vi "TLB Native Dynamic Events ver 0.26a.vi"() -> ()   [LabVIEW 2018] (continued)
          tunnel: w296 -> [_ _ _ _ _ _ _ _ _ _ _ _ _ _ _ _ _ _ _ _ _ _ _ _ _ _ _ _ _ _ _ _ _ _ _ _ _ _ _ _ w2086 _ _ _ _ _ _ _ w2455 _ _ _ _ _ _]
          tunnel: w295 -> [_ _ _ _ _ w505 _ _ _ _ _ _ _ _ w926 _ _ _ _ _ _ _ _ _ _ _ _ _ _ _ _ _ _ _ _ _ _ _ _ w2036 _ w2130 _ _ w2265 _ _ _ _ w2501 _ _ w2633 _ _]
          tunnel: [w337 w343 w360 w373 w492 w507 w552 w594 w640 w688 w734 w777 w823 w871 w927 w979 w1026 w1072 w1115 w1159 w1208 w1254 w1298 w1344 w1387 w1428 w1434 w1480 w1529 w1573 w1617 w1670 w1714 w1758 w1807 w1853 w1897 w1943 w1988 w2035 w2085 w2131 w2175 w2219 w2277 w2321 w2365 w2411 w2468 w2512 w2556 w2600 w2648 w2692 w2736] -> w293
          tunnel: w292 -> [w337 w343 w360 _ w492 w507 w552 w594 w640 w688 w734 w777 w823 w871 w927 w979 w1026 w1072 w1115 w1159 w1208 w1254 w1298 w1344 w1387 w1428 w1434 w1480 w1529 w1573 w1617 w1670 w1714 w1758 w1807 w1853 w1897 w1943 w1988 w2035 w2085 w2131 w2175 w2219 w2277 w2321 w2365 w2411 w2468 w2512 w2556 w2600 w2648 w2692 w2736]
          tunnel: w291 -> [_ _ _ _ _ _ _ _ _ _ _ _ _ _ _ _ _ _ _ _ _ _ _ _ _ _ _ _ _ _ _ _ _ _ _ _ _ _ _ _ w2084 _ _ _ _ _ _ _ _ _ _ _ _ _ _]
          tunnel: [_ _ _ _ _ _ _ _ w639 _ _ _ _ _ _ _ _ _ _ _ _ _ _ _ _ _ _ _ _ _ _ _ _ _ _ _ _ _ _ _ _ _ _ _ _ _ _ _ w2444 _ _ _ _ _ _] -> w290
          tunnel: [_ _ _ _ _ _ _ _ _ _ _ _ _ _ _ _ _ _ _ _ _ _ _ _ _ _ _ _ _ _ _ _ _ _ _ _ _ _ _ _ w2082 _ _ _ _ _ _ _ _ _ _ _ _ _ _] -> w289
          tunnel: [_ _ _ _ _ _ _ _ _ _ _ _ _ _ _ _ _ _ _ _ _ _ _ _ _ _ _ _ _ _ _ _ _ _ _ _ _ _ _ _ w2081 _ _ _ _ _ _ _ _ _ _ _ _ _ _] -> w288
          tunnel: w287 -> [_ _ _ _ _ _ _ _ _ _ _ _ _ _ _ _ _ _ _ _ _ _ _ _ _ _ _ _ _ _ _ _ _ _ _ _ _ _ _ _ _ _ _ _ _ _ _ _ _ _ _ _ _ _ _]
          frame 0 {
            # ">>> yStepper command>>>"
          }
          frame 1 {
            # ">>> yStepper command>>>"
            n201 = for {
              shift-right: [w359] -> w353
              shift-left: w356 -> [w358]
              tunnel: string[] ["INIT", "RESET ARM", "RESET FLAGS", "RESET YAW", "NAVX CALIBRATE"] -> [w357] mode=indexing
              n202 = Enqueue Element(queue=w358, element=w357) -> (queue out=w359:refnum<queue>)  [unwired: 2 in, 2 out]
            }
            n203 = Bundle By Name(cluster=w351, "yStepper desired"=u8 0) -> (w350:T20)
            n204 = Bundle By Name(cluster=w348, "ySpeed"=0.0, "xSpeed"=0.0, "wSpeed"=0.0) -> (w347:T19)
          }
          frame 3 {
            # ">>Action Queue>>"
            # ">>> Motor control cluster >>>"
            # ">>> yStepper command>>>"
            n205 = Flush Queue(queue=w366, error in (no error)=w365) -> ()  [unwired: 3 out]
            n206 = for {
              shift-right: [w372] -> w367
              shift-left: w368 -> [w371]
              tunnel: string[] ["STOP", "RESET ENCODERS", "RESET YAW", "RESET ARM", "RESET ALL SENSORS", "DISPOSE CAM BUFFERS", "DISPOSE PROC BUFFERS", "CAM CLOSE", ""] -> [w370] mode=indexing
              n207 = Enqueue Element(queue=w371, element=w370) -> (queue out=w372:refnum<queue>)  [unwired: 2 in, 2 out]
            }
          }
          frame 4, Default {
            # ">>> Motor control cluster >>>"
            # ">>> yStepper command>>>"
            n208 = Dequeue Element(queue=w384, timeout in ms (-1)=w383, error in (no error)=w379) -> (element=w382:T10)  [unwired: 3 out]
            n209 = case shown="\"Start Task 9\"" w382 {
              tunnel: [w387 w395 w403 w411 w419 w427 w435 w443 w451 w458 w468 w476 w483 w486] -> w378
              tunnel: w381 -> [w388 w396 w404 w412 w420 w428 w436 w444 w452 w459 w467 w475 w483 w487]
              tunnel: [State_Type_Definitions,_for_0.26g_versions_and_later_2."Task 1A" ("Enum") State_Type_Definitions,_for_0.26g_versions_and_later_2."Task 2:Raise Arm" ("Enum") State_Type_Definitions,_for_0.26g_versions_and_later_2."Task 3" ("Enum") State_Type_Definitions,_for_0.26g_versions_and_later_2."Task 4_A" ("Enum") State_Type_Definitions,_for_0.26g_versions_and_later_2."Task 5A" ("Enum") State_Type_Definitions,_for_0.26g_versions_and_later_2."Task 6_A" ("Enum") State_Type_Definitions,_for_0.26g_versions_and_later_2."Task 8A: RAISE ARM" ("Enum") State_Type_Definitions,_for_0.26g_versions_and_later_2."Task 8A: RAISE ARM" ("Enum") State_Type_Definitions,_for_0.26g_versions_and_later_2."Task 8A: RAISE ARM" ("Enum") State_Type_Definitions,_for_0.26g_versions_and_later_2."Task 8A: RAISE ARM" ("Enum") State_Type_Definitions,_for_0.26g_versions_and_later_2."Task 9A: Raise Arm" ("Enum") State_Type_Definitions."Task 9F: SCAN IMAGE" ("Enum") State_Type_Definitions,_for_0.26g_versions_and_later_2."Idle" ("Enum") State_Type_Definitions,_for_0.26g_versions_and_later_2."Shutdown" ("Enum")] -> w380
              tunnel: [enum16{"Ball", "Soap", "Gel", "Pipe", "None"}."None" ("Object recognition mode") enum16{"Ball", "Soap", "Gel", "Pipe", "None"}."None" ("Object recognition mode") enum16{"Ball", "Soap", "Gel", "Pipe", "None"}."None" ("Object recognition mode") enum16{"Ball", "Soap", "Gel", "Pipe", "None"}."None" ("Object recognition mode") enum16{"Ball", "Soap", "Gel", "Pipe", "None"}."None" ("Object recognition mode") enum16{"Ball", "Soap", "Gel", "Pipe", "None"}."None" ("Object recognition mode") enum16{"Ball", "Soap", "Gel", "Pipe", "None"}."Ball" ("Object recognition mode") enum16{"Ball", "Soap", "Gel", "Pipe", "None"}."Gel" ("Object recognition mode") enum16{"Ball", "Soap", "Gel", "Pipe", "None"}."Pipe" ("Object recognition mode") enum16{"Ball", "Soap", "Gel", "Pipe", "None"}."Soap" ("Object recognition mode") enum16{"Ball", "Soap", "Gel", "Pipe", "None"}."None" ("Object recognition mode") enum16{"Ball", "Soap", "Gel", "Pipe", "None"}."None" ("Object recognition mode") enum16{"Ball", "Soap", "Gel", "Pipe", "None"}."None" ("Object recognition mode") enum16{"Ball", "Soap", "Gel", "Pipe", "None"}."None" ("Object recognition mode")] -> w373
              frame "Start Task 1" {
                n210 = for {
                  shift-right: [w392] -> w387
                  shift-left: w388 -> [w391]
                  tunnel: string[] ["RESET ENCODERS", "RESET YAW", "FORWARD", "READ ENCODERS"] -> [w390] mode=indexing
                  n211 = Enqueue Element(queue=w391, element=w390) -> (queue out=w392:refnum<queue>)  [unwired: 2 in, 2 out]
                }
              }
              frame "Start Task 2" {
                n212 = for {
                  shift-right: [w400] -> w395
                  shift-left: w396 -> [w399]
                  tunnel: string[] ["RESET ENCODERS", "RESET YAW", "READ ULTRASONIC", "ARDUINO - ULTRASONIC"] -> [w398] mode=indexing
                  n213 = Enqueue Element(queue=w399, element=w398) -> (queue out=w400:refnum<queue>)  [unwired: 2 in, 2 out]
                }
              }
              frame "Start Task 3" {
                n214 = for {
                  shift-right: [w408] -> w403
                  shift-left: w404 -> [w407]
                  tunnel: string[] ["RESET ENCODERS", "READ ENCODERS", "R-ACW"] -> [w406] mode=indexing
                  n215 = Enqueue Element(queue=w407, element=w406) -> (queue out=w408:refnum<queue>)  [unwired: 2 in, 2 out]
                }
              }
              frame "Start Task 4" {
                n216 = for {
                  shift-right: [w416] -> w411
                  shift-left: w412 -> [w415]
                  tunnel: string[] ["RESET YAW", "RESET ENCODERS", "RESET ARM", "RESET FLAGS", "", ""] -> [w414] mode=indexing
                  n217 = Enqueue Element(queue=w415, element=w414) -> (queue out=w416:refnum<queue>)  [unwired: 2 in, 2 out]
                }
              }
              frame "Start Task 5" {
                n218 = for {
                  shift-right: [w424] -> w419
                  shift-left: w420 -> [w423]
                  tunnel: string[] ["RESET YAW", "RESET ENCODERS", "RESET ARM", "RESET ALL SENSORS", "", ""] -> [w422] mode=indexing
                  n219 = Enqueue Element(queue=w423, element=w422) -> (queue out=w424:refnum<queue>)  [unwired: 2 in, 2 out]
                }
              }
              frame "Start Task 6" {
                n220 = for {
                  shift-right: [w432] -> w427
                  shift-left: w428 -> [w431]
                  tunnel: string[] ["OPEN LOG CAM ", "", "", "", "", ""] -> [w430] mode=indexing
                  n221 = Enqueue Element(queue=w431, element=w430) -> (queue out=w432:refnum<queue>)  [unwired: 2 in, 2 out]
                }
              }
              frame "Start Task 8 - BALL" {
                n222 = for {
                  shift-right: [w440] -> w435
                  shift-left: w436 -> [w439]
                  tunnel: string[] ["RESET YAW", "RESET ENCODERS", "RESET ARM", "RESET FLAGS"] -> [w438] mode=indexing
                  n223 = Enqueue Element(queue=w439, element=w438) -> (queue out=w440:refnum<queue>)  [unwired: 2 in, 2 out]
                }
              }
              frame "Start Task 8 - Gel" {
                n224 = for {
                  shift-right: [w448] -> w443
                  shift-left: w444 -> [w447]
                  tunnel: string[] ["RESET YAW", "RESET ENCODERS", "RESET ARM", "RESET FLAGS"] -> [w446] mode=indexing
                  n225 = Enqueue Element(queue=w447, element=w446) -> (queue out=w448:refnum<queue>)  [unwired: 2 in, 2 out]
                }
              }
              frame "Start Task 8 - Pipe" {
                n226 = for {
                  shift-right: [w456] -> w451
                  shift-left: w452 -> [w455]
                  tunnel: string[] ["RESET YAW", "RESET ENCODERS", "RESET ARM", "RESET FLAGS"] -> [w454] mode=indexing
                  n227 = Enqueue Element(queue=w455, element=w454) -> (queue out=w456:refnum<queue>)  [unwired: 2 in, 2 out]
                }
              }
              frame "Start Task 8 - Soap" {
                n228 = for {
                  shift-right: [w464] -> w458
                  shift-left: w459 -> [w463]
                  tunnel: string[] ["RESET YAW", "RESET ENCODERS", "RESET ARM", "RESET FLAGS"] -> [w462] mode=indexing
                  n229 = Enqueue Element(queue=w463, element=w462) -> (queue out=w464:refnum<queue>)  [unwired: 2 in, 2 out]
                }
              }
              frame "Start Task 9" {
                n230 = for {
                  shift-right: [w472] -> w468
                  shift-left: w467 -> [w471]
                  tunnel: string[] ["RESET ENCODERS", "READ ENCODERS", "Z STEPPER BOX HEIGHT"] -> [w470] mode=indexing
                  n231 = Enqueue Element(queue=w471, element=w470) -> (queue out=w472:refnum<queue>)  [unwired: 2 in, 2 out]
                }
              }
              frame "Start Task A" {
                n232 = for {
                  shift-right: [w480] -> w476
                  shift-left: w475 -> [w479]
                  tunnel: string[] ["RESET ENCODERS", "READ ENCODERS", "RESET YAW", "Z STEPPER BOX HEIGHT"] -> [w478] mode=indexing
                  n233 = Enqueue Element(queue=w479, element=w478) -> (queue out=w480:refnum<queue>)  [unwired: 2 in, 2 out]
                }
              }
              frame "None", Default {
              }
              frame "Exit" {
                n234 = for {
                  shift-right: [w491] -> w486
                  shift-left: w487 -> [w490]
                  tunnel: string[] ["STOP", "RESET ENCODERS", "RESET YAW", "EXIT"] -> [w489] mode=indexing
                  n235 = Enqueue Element(queue=w490, element=w489) -> (queue out=w491:refnum<queue>)  [unwired: 2 in, 2 out]
                }
              }
            }
          }
          frame 5 {
            # ">> Item Selection Bias >>"
            # ">>> yStepper command>>>"
            n236 = for {
              shift-right: [w502] -> w496
              shift-left: w498 -> [w501]
              tunnel: string[] ["INIT", "RESET ENCODERS", "RESET FLAGS", "CAM CLOSE", "DISPOSE BUFFERS", "EXIT", ""] -> [w500] mode=indexing
              n237 = Enqueue Element(queue=w501, element=w500) -> (queue out=w502:refnum<queue>)  [unwired: 2 in, 2 out]
            }
          }
          frame 6 {
            # ">>> Motor control cluster >>>"
            # ">> Line detection >>"
            # ">> Checks if 1 metre moved >>"
            # ">>> yStepper command>>>"
            # "Use 250"
            n238 = Greater?(x=w512, y=265.0) -> (0:w506:bool)
            n239 = Dequeue Element(queue=w519, timeout in ms (-1)=w518, error in (no error)=w517) -> (element=w516:T10)  [unwired: 3 out]
            n240 = And(x=w505, y=w506) -> (x .and. y?=w503:bool)
            n241 = case shown="\"Start Task 1\", Default" w516 {
              tunnel: w504 -> [w520 _]
              tunnel: [w530 State_Type_Definitions,_for_0.26g_versions_and_later_2."True Stop" ("Enum")] -> w515
              tunnel: w514 -> [w528 w545]
              tunnel: [w527 w544] -> w513
              tunnel: [State_Type_Definitions,_for_0.26g_versions_and_later_2."Idle" ("Enum") State_Type_Definitions,_for_0.26g_versions_and_later_2."Shutdown" ("Enum")] -> w510
              tunnel: w503 -> [w521 _]
              frame "Start Task 1", Default {
                n242 = Or(x=w521, y=w520) -> (x .or. y?=w522:bool)
                n243 = case shown="True" w522 {
                  tunnel: w528 -> [w533 w539]
                  tunnel: [w532 w537] -> w527
                  frame False {
                    n244 = for {
                      shift-right: [w535] -> w532
                      shift-left: w533 -> [w536]
                      tunnel: string[] ["READ ENCODERS", "READ NAVX", "FORWARD", "READ LINE SENSOR"] ("element") -> [w534] mode=indexing
                      n245 = Enqueue Element(queue=w536, element=w534) -> (queue out=w535:refnum<queue>)  [unwired: 2 in, 2 out]
                    }
                  }
                  frame True {
                    n246 = for {
                      shift-right: [w541] -> w537
                      shift-left: w539 -> [w542]
                      tunnel: string[] ["RESET YAW", "RESET ENCODERS", "STOP", ""] -> [w540] mode=indexing
                      n247 = Enqueue Element(queue=w542, element=w540) -> (queue out=w541:refnum<queue>)  [unwired: 2 in, 2 out]
                    }
                  }
                }
                n248 = Select(t=State_Type_Definitions,_for_0.26g_versions_and_later_2."True Stop" ("Enum"), s=w520, f=State_Type_Definitions,_for_0.26g_versions_and_later_2."Task 1B" ("Enum")) -> (s? t:f=w525:T18)
                n249 = Select(t=w525, s=w521, f=State_Type_Definitions,_for_0.26g_versions_and_later_2."Task 1A" ("Enum")) -> (s? t:f=w530:T18)
              }
              frame "Exit" {
                n250 = for {
                  shift-right: [w549] -> w544
                  shift-left: w545 -> [w550]
                  tunnel: string[] ["STOP", "RESET ENCODERS", "RESET YAW", ""] -> [w548] mode=indexing
                  n251 = Enqueue Element(queue=w550, element=w548) -> (queue out=w549:refnum<queue>)  [unwired: 2 in, 2 out]
                }
              }
            }
          }
          frame 7 {
            # ">>> Motor control cluster >>>"
            # ">> Line detection >>"
            # ">> Adds small distance overhead after 1M >>"
            # ">>> yStepper command>>>"
            n252 = Greater?(x=w557, y=50.0) -> (0:w551:bool)
            n253 = Dequeue Element(queue=w566, timeout in ms (-1)=w565, error in (no error)=w564) -> (element=w563:T10)  [unwired: 3 out]
            n254 = Or(x=w551, y=w558) -> (x .or. y?=w562:bool)
            n255 = case shown="\"Start Task 1\", Default" w563 {
              tunnel: w562 -> [w569 _]
              tunnel: [w573 State_Type_Definitions,_for_0.26g_versions_and_later_2."True Stop" ("Enum")] -> w561
              tunnel: w560 -> [w570 w588]
              tunnel: [w568 w587] -> w559
              tunnel: [State_Type_Definitions,_for_0.26g_versions_and_later_2."Idle" ("Enum") State_Type_Definitions,_for_0.26g_versions_and_later_2."Shutdown" ("Enum")] -> w555
              frame "Start Task 1", Default {
                n256 = case shown="True" w569 {
                  tunnel: w570 -> [w576 w582]
                  tunnel: [w575 w580] -> w568
                  frame False {
                    n257 = for {
                      shift-right: [w578] -> w575
                      shift-left: w576 -> [w579]
                      tunnel: string[] ["READ ENCODERS", "READ NAVX", "FORWARD", "READ LINE SENSOR"] ("element") -> [w577] mode=indexing
                      n258 = Enqueue Element(queue=w579, element=w577) -> (queue out=w578:refnum<queue>)  [unwired: 2 in, 2 out]
                    }
                  }
                  frame True {
                    n259 = for {
                      shift-right: [w584] -> w580
                      shift-left: w582 -> [w585]
                      tunnel: string[] ["RESET YAW", "RESET ENCODERS", "STOP", ""] -> [w583] mode=indexing
                      n260 = Enqueue Element(queue=w585, element=w583) -> (queue out=w584:refnum<queue>)  [unwired: 2 in, 2 out]
                    }
                  }
                }
                n261 = Select(t=State_Type_Definitions,_for_0.26g_versions_and_later_2."True Stop" ("Enum"), s=w569, f=State_Type_Definitions,_for_0.26g_versions_and_later_2."Task 1B" ("Enum")) -> (s? t:f=w573:T18)
              }
              frame "Exit" {
                n262 = for {
                  shift-right: [w592] -> w587
                  shift-left: w588 -> [w593]
                  tunnel: string[] ["STOP", "RESET ENCODERS", "RESET YAW", ""] -> [w591] mode=indexing
                  n263 = Enqueue Element(queue=w593, element=w591) -> (queue out=w592:refnum<queue>)  [unwired: 2 in, 2 out]
                }
              }
            }
          }
          frame 8 {
            # ">> Stepper height reeached >>"
            # ">>> yStepper command>>>"
            # ">> Manual override >>"
            n264 = Dequeue Element(queue=w599, timeout in ms (-1)=w598, error in (no error)=w597) -> (element=w608:T10)  [unwired: 3 out]
            n265 = Equal?(x=w601, y=u8 60) -> (x = y?=w606:bool)
            n266 = case shown="\"Start Task 1\", Default" w608 {
              tunnel: [w619 State_Type_Definitions,_for_0.26g_versions_and_later_2."True Stop" ("Enum")] -> w603
              tunnel: [w617 w634] -> w596
              tunnel: w605 -> [w616 _]
              tunnel: w604 -> [w610 _]
              tunnel: [State_Type_Definitions,_for_0.26g_versions_and_later_2."Idle" ("Enum") State_Type_Definitions,_for_0.26g_versions_and_later_2."Shutdown" ("Enum")] -> w602
              tunnel: w606 -> [w609 _]
              frame "Start Task 1", Default {
                # ">> WIill proceed to part ii if not manual override >>"
                # ">>If ENABLE or Trigger is set to true>>"
                n267 = Or(x=w609, y=w610) -> (x .or. y?=w611:bool)
                n268 = case shown="True" w609 {
                  tunnel: [w622 w628] -> w617
                  tunnel: w616 -> [w621 w627]
                  frame False {
                    n269 = for {
                      shift-right: [w624] -> w622
                      shift-left: w621 -> [w625]
                      tunnel: string[] ["Z STEPPER CAM HEIGHT", "READ STEPPER VALUES"] ("element") -> [w623] mode=indexing
                      n270 = Enqueue Element(queue=w625, element=w623) -> (queue out=w624:refnum<queue>)  [unwired: 2 in, 2 out]
                    }
                  }
                  frame True {
                    n271 = for {
                      shift-right: [w630] -> w628
                      shift-left: w627 -> [w631]
                      tunnel: string[] ["ARDUINO - ULTRASONIC", "READ ULTRASONIC", "", "", "", ""] -> [w629] mode=indexing
                      n272 = Enqueue Element(queue=w631, element=w629) -> (queue out=w630:refnum<queue>)  [unwired: 2 in, 2 out]
                    }
                  }
                }
                n273 = Select(t=State_Type_Definitions,_for_0.26g_versions_and_later_2."True Stop" ("Enum"), s=w610, f=State_Type_Definitions,_for_0.26g_versions_and_later_2."Task 2:Sensor Mode" ("Enum")) -> (s? t:f=w613:T18)
                n274 = Select(t=w613, s=w611, f=State_Type_Definitions,_for_0.26g_versions_and_later_2."Task 2:Raise Arm" ("Enum")) -> (s? t:f=w619:T18)
              }
              frame "Exit" {
                n275 = for {
                  shift-right: [w637] -> w634
                  shift-left: _ -> [w638]
                  tunnel: string[] ["STOP", "RESET ENCODERS", "RESET YAW", ""] -> [w636] mode=indexing
                  n276 = Enqueue Element(queue=w638, element=w636) -> (queue out=w637:refnum<queue>)  [unwired: 2 in, 2 out]
                }
              }
            }
          }
          frame 9 {
            w655 = u8 20 ("y")
            # ">>> yStepper command>>>"
            # ">>Object detected>>"
            n277 = Dequeue Element(queue=w648, timeout in ms (-1)=w647, error in (no error)=w646) -> (element=w656:T10)  [unwired: 3 out]
            n278 = Less?(x=w644, y=w655) -> (x < y?=w654:bool)
            n279 = Less?(x=w643, y=w655) -> (x < y?=w653:bool)
            n280 = Or(x=w654, y=w653) -> (x .or. y?=w639:bool)
            n281 = case shown="\"Start Task 1\", Default" w656 {
              tunnel: w639 -> [w659 _]
              tunnel: [w666 State_Type_Definitions,_for_0.26g_versions_and_later_2."True Stop" ("Enum")] -> w652
              tunnel: w645 -> [w658 _]
              tunnel: w649 -> [w665 w682]
              tunnel: [w664 w683] -> w651
              tunnel: [State_Type_Definitions,_for_0.26g_versions_and_later_2."Idle" ("Enum") State_Type_Definitions,_for_0.26g_versions_and_later_2."Shutdown" ("Enum")] -> w650
              frame "Start Task 1", Default {
                n282 = case shown="False" w659 {
                  tunnel: w665 -> [w669 w676]
                  tunnel: [w670 w675] -> w664
                  frame False {
                    n283 = for {
                      tunnel: string[] ["READ ULTRASONIC", "STOP"] ("element") -> [w671] mode=indexing
                      shift-right: [w673] -> w670
                      shift-left: w669 -> [w672]
                      n284 = Enqueue Element(queue=w672, element=w671) -> (queue out=w673:refnum<queue>)  [unwired: 2 in, 2 out]
                    }
                  }
                  frame True {
                    n285 = for {
                      shift-right: [w678] -> w675
                      shift-left: w676 -> [w679]
                      tunnel: string[] ["RESET ENCODERS", "READ NAVX", "READ ENCODERS"] -> [w677] mode=indexing
                      n286 = Enqueue Element(queue=w679, element=w677) -> (queue out=w678:refnum<queue>)  [unwired: 2 in, 2 out]
                    }
                  }
                }
                n287 = Or(x=w659, y=w658) -> (x .or. y?=w657:bool)
                n288 = Select(t=State_Type_Definitions,_for_0.26g_versions_and_later_2."True Stop" ("Enum"), s=w658, f=State_Type_Definitions,_for_0.26g_versions_and_later_2."Task 2:Reverse Mode" ("Enum")) -> (s? t:f=w660:T18)
                n289 = Select(t=w660, s=w657, f=State_Type_Definitions,_for_0.26g_versions_and_later_2."Task 2:Sensor Mode" ("Enum")) -> (s? t:f=w666:T18)
              }
              frame "Exit" {
                n290 = for {
                  shift-right: [w686] -> w683
                  shift-left: w682 -> [w687]
                  tunnel: string[] ["STOP", "RESET ENCODERS", "RESET YAW", "ARDUINO MODE 0"] -> [w685] mode=indexing
                  n291 = Enqueue Element(queue=w687, element=w685) -> (queue out=w686:refnum<queue>)  [unwired: 2 in, 2 out]
                }
              }
            }
          }
          frame 10 {
            # ">>> yStepper command>>>"
            n292 = Dequeue Element(queue=w698, timeout in ms (-1)=w699, error in (no error)=w700) -> (element=w702:T10)  [unwired: 3 out]
            n293 = Less?(x=w692, y=-50.0) -> (x < y?=w690:bool)
            n294 = case shown="\"Start Task 1\", Default" w702 {
              tunnel: [w712 State_Type_Definitions,_for_0.26g_versions_and_later_2."True Stop" ("Enum")] -> w694
              tunnel: w701 -> [w705 _]
              tunnel: w697 -> [w711 w728]
              tunnel: [w710 w729] -> w693
              tunnel: [State_Type_Definitions,_for_0.26g_versions_and_later_2."Idle" ("Enum") State_Type_Definitions,_for_0.26g_versions_and_later_2."Shutdown" ("Enum")] -> w695
              tunnel: w690 -> [w703 _]
              frame "Start Task 1", Default {
                n295 = case shown="True" w703 {
                  tunnel: w711 -> [w715 w722]
                  tunnel: [w716 w721] -> w710
                  frame False {
                    n296 = for {
                      tunnel: string[] ["READ ENCODERS", "REVERSE", "READ NAVX"] ("element") -> [w717] mode=indexing
                      shift-right: [w719] -> w716
                      shift-left: w715 -> [w718]
                      n297 = Enqueue Element(queue=w718, element=w717) -> (queue out=w719:refnum<queue>)  [unwired: 2 in, 2 out]
                    }
                  }
                  frame True {
                    n298 = for {
                      shift-right: [w724] -> w721
                      shift-left: w722 -> [w725]
                      tunnel: string[] ["STOP", "ARDUINO - ULTRASONIC", "READ ULTRASONIC", "RESET ENCODERS"] -> [w723] mode=indexing
                      n299 = Enqueue Element(queue=w725, element=w723) -> (queue out=w724:refnum<queue>)  [unwired: 2 in, 2 out]
                    }
                  }
                }
                n300 = Or(x=w703, y=w705) -> (x .or. y?=w704:bool)
                n301 = Select(t=State_Type_Definitions,_for_0.26g_versions_and_later_2."True Stop" ("Enum"), s=w705, f=State_Type_Definitions,_for_0.26g_versions_and_later_2."Task 2:Sensor Mode" ("Enum")) -> (s? t:f=w706:T18)
                n302 = Select(t=w706, s=w704, f=State_Type_Definitions,_for_0.26g_versions_and_later_2."Task 2:Reverse Mode" ("Enum")) -> (s? t:f=w712:T18)
              }
              frame "Exit" {
                n303 = for {
                  shift-right: [w732] -> w729
                  shift-left: w728 -> [w733]
                  tunnel: string[] ["STOP", "RESET ENCODERS", "RESET YAW", "ARDUINO MODE 0"] -> [w731] mode=indexing
                  n304 = Enqueue Element(queue=w733, element=w731) -> (queue out=w732:refnum<queue>)  [unwired: 2 in, 2 out]
                }
              }
            }
          }
          frame 11 {
            # ">>> Motor control cluster >>>"
            # ">>> yStepper command>>>"
            n305 = Dequeue Element(queue=w749, timeout in ms (-1)=w748, error in (no error)=w747) -> (element=w738:T10)  [unwired: 3 out]
            n306 = Less?(x=w746, y=-160.0) -> (x < y?=w743:bool)
            n307 = Or(x=w743, y=w744) -> (x .or. y?=w739:bool)
            n308 = case shown="\"Start Task 1\", Default" w738 {
              tunnel: w739 -> [w752 _]
              tunnel: [w756 State_Type_Definitions,_for_0.26g_versions_and_later_2."True Stop" ("Enum")] -> w740
              tunnel: w742 -> [w753 w772]
              tunnel: [w751 w771] -> w741
              tunnel: [State_Type_Definitions,_for_0.26g_versions_and_later_2."Idle" ("Enum") State_Type_Definitions,_for_0.26g_versions_and_later_2."Shutdown" ("Enum")] -> w737
              frame "Start Task 1", Default {
                n309 = case shown="False" w752 {
                  tunnel: w753 -> [w759 w765]
                  tunnel: [w758 w763] -> w751
                  frame False {
                    n310 = for {
                      shift-right: [w761] -> w758
                      shift-left: w759 -> [w762]
                      tunnel: string[] ["READ ENCODERS", "R-CW"] ("element") -> [w760] mode=indexing
                      n311 = Enqueue Element(queue=w762, element=w760) -> (queue out=w761:refnum<queue>)  [unwired: 2 in, 2 out]
                    }
                  }
                  frame True {
                    n312 = for {
                      shift-right: [w767] -> w763
                      shift-left: w765 -> [w768]
                      tunnel: string[] ["RESET YAW", "RESET ENCODERS", "STOP", "ARDUINO MODE 0"] -> [w766] mode=indexing
                      n313 = Enqueue Element(queue=w768, element=w766) -> (queue out=w767:refnum<queue>)  [unwired: 2 in, 2 out]
                    }
                  }
                }
                n314 = Select(t=State_Type_Definitions,_for_0.26g_versions_and_later_2."True Stop" ("Enum"), s=w752, f=State_Type_Definitions,_for_0.26g_versions_and_later_2."Task 3" ("Enum")) -> (s? t:f=w756:T18)
              }
              frame "Exit" {
                n315 = for {
                  shift-right: [w775] -> w771
                  shift-left: w772 -> [w776]
                  tunnel: string[] ["STOP", "RESET ENCODERS", "RESET YAW", ""] -> [w774] mode=indexing
                  n316 = Enqueue Element(queue=w776, element=w774) -> (queue out=w775:refnum<queue>)  [unwired: 2 in, 2 out]
                }
              }
            }
          }
          frame 12 {
            # ">> Stepper height reeached >>"
            # ">>> yStepper command>>>"
            # ">> Manual override >>"
            n317 = Dequeue Element(queue=w790, timeout in ms (-1)=w789, error in (no error)=w788) -> (element=w787:T10)  [unwired: 3 out]
            n318 = Equal?(x=w781, y=u8 60) -> (x = y?=w779:bool)
            n319 = case shown="\"Start Task 1\", Default" w787 {
              tunnel: [w802 State_Type_Definitions,_for_0.26g_versions_and_later_2."True Stop" ("Enum")] -> w786
              tunnel: [w800 w818] -> w785
              tunnel: w791 -> [w799 w815]
              tunnel: w784 -> [w793 _]
              tunnel: [State_Type_Definitions,_for_0.26g_versions_and_later_2."Idle" ("Enum") State_Type_Definitions,_for_0.26g_versions_and_later_2."Shutdown" ("Enum")] -> w783
              tunnel: w779 -> [w792 _]
              frame "Start Task 1", Default {
                # ">> WIill proceed to part ii if not manual override >>"
                # ">>If ENABLE or Trigger is set to true>>"
                n320 = Or(x=w792, y=w793) -> (x .or. y?=w794:bool)
                n321 = case shown="False" w792 {
                  tunnel: [w805 w811] -> w800
                  tunnel: w799 -> [w804 w810]
                  frame False {
                    n322 = for {
                      shift-right: [w807] -> w805
                      shift-left: w804 -> [w808]
                      tunnel: string[] ["Z STEPPER CAM HEIGHT", "READ STEPPER VALUES"] ("element") -> [w806] mode=indexing
                      n323 = Enqueue Element(queue=w808, element=w806) -> (queue out=w807:refnum<queue>)  [unwired: 2 in, 2 out]
                    }
                  }
                  frame True {
                    n324 = for {
                      shift-right: [w813] -> w811
                      shift-left: w810 -> [w814]
                      tunnel: string[] ["ARDUINO - ULTRASONIC", "READ ULTRASONIC", "FORWARD", "", "", ""] -> [w812] mode=indexing
                      n325 = Enqueue Element(queue=w814, element=w812) -> (queue out=w813:refnum<queue>)  [unwired: 2 in, 2 out]
                    }
                  }
                }
                n326 = Select(t=State_Type_Definitions,_for_0.26g_versions_and_later_2."True Stop" ("Enum"), s=w793, f=State_Type_Definitions,_for_0.26g_versions_and_later_2."Task 4_B" ("Enum")) -> (s? t:f=w796:T18)
                n327 = Select(t=w796, s=w794, f=State_Type_Definitions,_for_0.26g_versions_and_later_2."Task 4_A" ("Enum")) -> (s? t:f=w802:T18)
              }
              frame "Exit" {
                n328 = for {
                  shift-right: [w821] -> w818
                  shift-left: w815 -> [w822]
                  tunnel: string[] ["STOP", "RESET ENCODERS", "RESET YAW", ""] -> [w820] mode=indexing
                  n329 = Enqueue Element(queue=w822, element=w820) -> (queue out=w821:refnum<queue>)  [unwired: 2 in, 2 out]
                }
              }
            }
          }
          frame 13 {
            w828 = u8 20
            # ">> Path blocked >>"
            # ">>> yStepper command>>>"
            # ">> Manual override >>"
            n330 = Dequeue Element(queue=w837, timeout in ms (-1)=w836, error in (no error)=w835) -> (element=w834:T10)  [unwired: 3 out]
            n331 = Less?(x=w830, y=w828) -> (x < y?=w825:bool)
            n332 = Less?(x=w829, y=w828) -> (x < y?=w826:bool)
            n333 = And(x=w826, y=w825) -> (x .and. y?=w827:bool)
            n334 = case shown="\"Start Task 1\", Default" w834 {
              tunnel: [w851 State_Type_Definitions,_for_0.26g_versions_and_later_2."True Stop" ("Enum")] -> w839
              tunnel: [w849 w866] -> w840
              tunnel: w833 -> [w848 _]
              tunnel: w838 -> [w842 _]
              tunnel: [State_Type_Definitions,_for_0.26g_versions_and_later_2."Idle" ("Enum") State_Type_Definitions,_for_0.26g_versions_and_later_2."Shutdown" ("Enum")] -> w832
              tunnel: w827 -> [w841 _]
              frame "Start Task 1", Default {
                # ">> Manual override forces program to true stop >>"
                # ">>If ENABLE or Trigger is set to true>>"
                n335 = Or(x=w841, y=w842) -> (x .or. y?=w847:bool)
                n336 = case shown="False" w841 {
                  tunnel: [w854 w859] -> w849
                  tunnel: w848 -> [w853 w858]
                  frame False {
                    n337 = for {
                      shift-right: [w856] -> w854
                      shift-left: w853 -> [w857]
                      tunnel: string[] ["FORWARD", "READ ULTRASONIC", "READ NAVX"] ("element") -> [w855] mode=indexing
                      n338 = Enqueue Element(queue=w857, element=w855) -> (queue out=w856:refnum<queue>)  [unwired: 2 in, 2 out]
                    }
                  }
                  frame True {
                    n339 = for {
                      shift-right: [w862] -> w859
                      shift-left: w858 -> [w863]
                      tunnel: string[] ["STOP", "RESET YAW", "RESET ENCODERS", "RESET FLAGS"] -> [w861] mode=indexing
                      n340 = Enqueue Element(queue=w863, element=w861) -> (queue out=w862:refnum<queue>)  [unwired: 2 in, 2 out]
                    }
                  }
                }
                n341 = Select(t=State_Type_Definitions,_for_0.26g_versions_and_later_2."True Stop" ("Enum"), s=w842, f=State_Type_Definitions,_for_0.26g_versions_and_later_2."Task 4_C" ("Enum")) -> (s? t:f=w844:T18)
                n342 = Select(t=w844, s=w847, f=State_Type_Definitions,_for_0.26g_versions_and_later_2."Task 4_B" ("Enum")) -> (s? t:f=w851:T18)
              }
              frame "Exit" {
                n343 = for {
                  shift-right: [w869] -> w866
                  shift-left: _ -> [w870]
                  tunnel: string[] ["STOP", "RESET ENCODERS", "RESET YAW", ""] -> [w868] mode=indexing
                  n344 = Enqueue Element(queue=w870, element=w868) -> (queue out=w869:refnum<queue>)  [unwired: 2 in, 2 out]
                }
              }
            }
          }
          frame 14 {
            w882 = u8 20
            # ">> xDistance travelled>>"
            # ">> Path NOT blocked >>"
            # ">>> yStepper command>>>"
            # ">> Manual override >>"
            n345 = Dequeue Element(queue=w892, timeout in ms (-1)=w885, error in (no error)=w884) -> (element=w886:T10)  [unwired: 3 out]
            n346 = Greater?(x=w874, y=w882) -> (0:w880:bool)
            n347 = Greater?(x=w879, y=80.0) -> (0:w877:bool)
            n348 = Greater?(x=w873, y=w882) -> (0:w881:bool)
            n349 = And(x=w881, y=w880) -> (x .and. y?=w876:bool)
            n350 = And(x=w877, y=w876) -> (x .and. y?=w875:bool)
            n351 = case shown="\"Start Task 1\", Default" w886 {
              tunnel: [w903 State_Type_Definitions,_for_0.26g_versions_and_later_2."True Stop" ("Enum")] -> w889
              tunnel: [w901 w919] -> w888
              tunnel: w891 -> [w900 w916]
              tunnel: w890 -> [w894 _]
              tunnel: [State_Type_Definitions,_for_0.26g_versions_and_later_2."Idle" ("t") State_Type_Definitions,_for_0.26g_versions_and_later_2."Shutdown" ("Enum")] -> w887
              tunnel: w875 -> [w893 _]
              frame "Start Task 1", Default {
                # ">> Manual override forces program to true stop >>"
                # ">>If ENABLE or Trigger is set to true>>"
                n352 = Or(x=w893, y=w894) -> (x .or. y?=w899:bool)
                n353 = case shown="False" w893 {
                  tunnel: [w906 w911] -> w901
                  tunnel: w900 -> [w904 w910]
                  frame False {
                    n354 = for {
                      shift-right: [w908] -> w906
                      shift-left: w904 -> [w909]
                      tunnel: string[] ["RIGHT", "READ NAVX", "READ ENCODERS", "READ ULTRASONIC"] ("element") -> [w907] mode=indexing
                      n355 = Enqueue Element(queue=w909, element=w907) -> (queue out=w908:refnum<queue>)  [unwired: 2 in, 2 out]
                    }
                  }
                  frame True {
                    n356 = for {
                      shift-right: [w914] -> w911
                      shift-left: w910 -> [w915]
                      tunnel: string[] ["STOP", "RESET YAW", "RESET ENCODERS", "ARDUINO - ULTRASONIC"] -> [w913] mode=indexing
                      n357 = Enqueue Element(queue=w915, element=w913) -> (queue out=w914:refnum<queue>)  [unwired: 2 in, 2 out]
                    }
                  }
                }
                n358 = Select(t=State_Type_Definitions,_for_0.26g_versions_and_later_2."True Stop" ("Enum"), s=w894, f=State_Type_Definitions,_for_0.26g_versions_and_later_2."Task 4_D" ("Enum")) -> (s? t:f=w895:T18)
                n359 = Select(t=w895, s=w899, f=State_Type_Definitions,_for_0.26g_versions_and_later_2."Task 4_C" ("Enum")) -> (s? t:f=w903:T18)
              }
              frame "Exit" {
                n360 = for {
                  shift-right: [w922] -> w919
                  shift-left: w916 -> [w923]
                  tunnel: string[] ["STOP", "RESET ENCODERS", "RESET YAW", ""] -> [w921] mode=indexing
                  n361 = Enqueue Element(queue=w923, element=w921) -> (queue out=w922:refnum<queue>)  [unwired: 2 in, 2 out]
                }
              }
            }
          }
          frame 15 {
            w946 = u8 20
            # ">>> Motor control cluster >>>"
            # ">> Line detected >>"
            # ">> yDistance travelled>>"
            # ">> Path blocked >>"
            # ">>> yStepper command>>>"
            # ">> Manual override >>"
            n362 = Less?(x=w931, y=w946) -> (x < y?=w944:bool)
            n363 = Greater?(x=w935, y=200.0) -> (0:w942:bool)
            n364 = Less?(x=w930, y=w946) -> (x < y?=w945:bool)
            n365 = And(x=w945, y=w944) -> (x .and. y?=w941:bool)
            n366 = Dequeue Element(queue=w938, timeout in ms (-1)=w937, error in (no error)=w936) -> (element=w947:T10)  [unwired: 3 out]
            n367 = Or(x=w942, y=w941) -> (x .or. y?=w925:bool)
            n368 = And(x=w926, y=w925) -> (x .and. y?=w924:bool)
            n369 = case shown="\"Start Task 1\", Default" w947 {
              tunnel: [w958 State_Type_Definitions,_for_0.26g_versions_and_later_2."True Stop" ("Enum")] -> w934
              tunnel: [w956 w974] -> w932
              tunnel: w939 -> [w955 w971]
              tunnel: w940 -> [w949 _]
              tunnel: [State_Type_Definitions,_for_0.26g_versions_and_later_2."Idle" ("t") State_Type_Definitions,_for_0.26g_versions_and_later_2."Shutdown" ("Enum")] -> w933
              tunnel: w924 -> [w948 _]
              frame "Start Task 1", Default {
                # ">> Manual override forces program to true stop >>"
                # ">>If ENABLE or Trigger is set to true>>"
                n370 = Or(x=w948, y=w949) -> (x .or. y?=w954:bool)
                n371 = case shown="False" w948 {
                  tunnel: [w961 w966] -> w956
                  tunnel: w955 -> [w959 w965]
                  frame False {
                    n372 = for {
                      shift-right: [w963] -> w961
                      shift-left: w959 -> [w964]
                      tunnel: string[] ["FORWARD", "READ NAVX", "READ ENCODERS", "READ ULTRASONIC", "READ LINE SENSOR"] ("element") -> [w962] mode=indexing
                      n373 = Enqueue Element(queue=w964, element=w962) -> (queue out=w963:refnum<queue>)  [unwired: 2 in, 2 out]
                    }
                  }
                  frame True {
                    n374 = for {
                      shift-right: [w969] -> w966
                      shift-left: w965 -> [w970]
                      tunnel: string[] ["STOP", "RESET YAW", "RESET ENCODERS", "RESET FLAGS"] -> [w968] mode=indexing
                      n375 = Enqueue Element(queue=w970, element=w968) -> (queue out=w969:refnum<queue>)  [unwired: 2 in, 2 out]
                    }
                  }
                }
                n376 = Select(t=State_Type_Definitions,_for_0.26g_versions_and_later_2."True Stop" ("Enum"), s=w949, f=State_Type_Definitions,_for_0.26g_versions_and_later_2."True Stop" ("Enum")) -> (s? t:f=w950:T18)
                n377 = Select(t=w950, s=w954, f=State_Type_Definitions,_for_0.26g_versions_and_later_2."Task 4_D" ("Enum")) -> (s? t:f=w958:T18)
              }
              frame "Exit" {
                n378 = for {
                  shift-right: [w977] -> w974
                  shift-left: w971 -> [w978]
                  tunnel: string[] ["STOP", "RESET ENCODERS", "RESET YAW", ""] -> [w976] mode=indexing
                  n379 = Enqueue Element(queue=w978, element=w976) -> (queue out=w977:refnum<queue>)  [unwired: 2 in, 2 out]
                }
              }
            }
          }
          frame 16 {
            # "Stays in Task 5_A until stepper reaches desired \nheight"
            # ">>> Motor control cluster >>>"
            # ">>> yStepper command>>>"
            # ">> Manual override >>"
            n380 = Dequeue Element(queue=w989, timeout in ms (-1)=w988, error in (no error)=w990) -> (element=w987:T10)  [unwired: 3 out]
            n381 = Equal?(x=w986, y=u8 1) -> (x = y?=w984:bool)
            n382 = case shown="\"Start Task 1\", Default" w987 {
              tunnel: [w1000 State_Type_Definitions,_for_0.26g_versions_and_later_2."True Stop" ("Enum")] -> w991
              tunnel: [w1003 w1020] -> w992
              tunnel: [State_Type_Definitions,_for_0.26g_versions_and_later_2."Idle" ("Enum") State_Type_Definitions,_for_0.26g_versions_and_later_2."Shutdown" ("Enum")] -> w993
              tunnel: w984 -> [w999 _]
              tunnel: w983 -> [w998 _]
              tunnel: w982 -> [w994 w1017]
              frame "Start Task 1", Default {
                # "T: Go back to idle, F: Continue with task\""
                # ">> Manual override >>"
                n383 = case shown="True" w999 {
                  tunnel: [w1007 w1013] -> w1003
                  tunnel: w994 -> [w1005 w1011]
                  frame False {
                    n384 = for {
                      tunnel: string[] ["Z STEPPER GRAB HEIGHT", "READ STEPPER VALUES"] ("element") -> [w1008] mode=indexing
                      shift-right: [w1010] -> w1007
                      shift-left: w1005 -> [w1009]
                      n385 = Enqueue Element(queue=w1009, element=w1008) -> (queue out=w1010:refnum<queue>)  [unwired: 2 in, 2 out]
                    }
                  }
                  frame True {
                    n386 = for {
                      shift-right: [w1015] -> w1013
                      shift-left: w1011 -> [w1016]
                      tunnel: string[] ["SET TIMER 2", "", ""] -> [w1014] mode=indexing
                      n387 = Enqueue Element(queue=w1016, element=w1014) -> (queue out=w1015:refnum<queue>)  [unwired: 2 in, 2 out]
                    }
                  }
                }
                n388 = Or(x=w999, y=w998) -> (x .or. y?=w1001:bool)
                n389 = Select(t=State_Type_Definitions,_for_0.26g_versions_and_later_2."True Stop" ("Enum"), s=w998, f=State_Type_Definitions,_for_0.26g_versions_and_later_2."Task 5B" ("Enum")) -> (s? t:f=w995:T18)
                n390 = Select(t=w995, s=w1001, f=State_Type_Definitions,_for_0.26g_versions_and_later_2."Task 5A" ("Enum")) -> (s? t:f=w1000:T18)
              }
              frame "Exit" {
                n391 = for {
                  shift-right: [w1023] -> w1020
                  shift-left: w1017 -> [w1024]
                  tunnel: string[] ["STOP", "RESET ENCODERS", "RESET YAW", "ARDUINO MODE 0"] -> [w1022] mode=indexing
                  n392 = Enqueue Element(queue=w1024, element=w1022) -> (queue out=w1023:refnum<queue>)  [unwired: 2 in, 2 out]
                }
              }
            }
          }
          frame 17 {
            # ">>> yStepper command>>>"
            n393 = Dequeue Element(queue=w1031, timeout in ms (-1)=w1030, error in (no error)=w1032) -> (element=w1029:T10)  [unwired: 3 out]
            n394 = case shown="\"Start Task 1\", Default" w1029 {
              tunnel: [w1044 State_Type_Definitions,_for_0.26g_versions_and_later_2."True Stop" ("Enum")] -> w1034
              tunnel: [w1047 w1064] -> w1033
              tunnel: [State_Type_Definitions,_for_0.26g_versions_and_later_2."Idle" ("Enum") State_Type_Definitions,_for_0.26g_versions_and_later_2."Shutdown" ("Enum")] -> w1035
              tunnel: w1037 -> [w1043 _]
              tunnel: w1036 -> [w1039 w1061]
              tunnel: w1025 -> [w1038 _]
              frame "Start Task 1", Default {
                # "T: Go back to idle, F: Continue with task\""
                # ">> Manual override >>"
                n395 = case shown="True" w1038 {
                  tunnel: [w1051 w1057] -> w1047
                  tunnel: w1039 -> [w1049 w1055]
                  frame False {
                    n396 = for {
                      tunnel: string[] ["CLOSE CLAW", "START TIMER", ""] ("element") -> [w1052] mode=indexing
                      shift-right: [w1054] -> w1051
                      shift-left: w1049 -> [w1053]
                      n397 = Enqueue Element(queue=w1053, element=w1052) -> (queue out=w1054:refnum<queue>)  [unwired: 2 in, 2 out]
                    }
                  }
                  frame True {
                    n398 = for {
                      shift-right: [w1059] -> w1057
                      shift-left: w1055 -> [w1060]
                      tunnel: string[] ["STOP", "", "", ""] -> [w1058] mode=indexing
                      n399 = Enqueue Element(queue=w1060, element=w1058) -> (queue out=w1059:refnum<queue>)  [unwired: 2 in, 2 out]
                    }
                  }
                }
                n400 = Or(x=w1038, y=w1043) -> (x .or. y?=w1045:bool)
                n401 = Select(t=State_Type_Definitions,_for_0.26g_versions_and_later_2."True Stop" ("Enum"), s=w1043, f=State_Type_Definitions,_for_0.26g_versions_and_later_2."Task 5C" ("Enum")) -> (s? t:f=w1040:T18)
                n402 = Select(t=w1040, s=w1045, f=State_Type_Definitions,_for_0.26g_versions_and_later_2."Task 5B" ("Enum")) -> (s? t:f=w1044:T18)
              }
              frame "Exit" {
                n403 = for {
                  shift-right: [w1067] -> w1064
                  shift-left: w1061 -> [w1068]
                  tunnel: string[] ["STOP", "RESET ENCODERS", "RESET YAW", "ARDUINO MODE 0"] -> [w1066] mode=indexing
                  n404 = Enqueue Element(queue=w1068, element=w1066) -> (queue out=w1067:refnum<queue>)  [unwired: 2 in, 2 out]
                }
              }
            }
          }
          frame 18 {
            # ">>> Motor control cluster >>>"
            # ">>> yStepper command>>>"
            # ">> Manual override >>"
            n405 = Equal?(x=w1071, y=u8 60) -> (x = y?=w1069:bool)
            n406 = Dequeue Element(queue=w1081, timeout in ms (-1)=w1080, error in (no error)=w1079) -> (element=w1078:T10)  [unwired: 3 out]
            n407 = case shown="\"Start Task 1\", Default" w1078 {